vi "UHR-Fleezers Control (host) - 12.7c.vi"() -> ()   [LabVIEW 2012] (continued)
      }
      event "Abort AOD Scan": Value Change {
        n1196 = event-data() -> ()  [unwired: 7 out]
        n1197 = xnode "Read/Write Control"("FPGA VI Reference In"=w1678, "error in"=w1677, "Abort scan"="Abort AOD Scan") -> ("error out"=w1676:errorcluster)  [unwired: 1 out]
      }
      event "Continuous AOD Scanning": Value Change {
        n1198 = event-data() -> ()  [unwired: 7 out]
        n1199 = xnode "Read/Write Control"("FPGA VI Reference In"=w1682, "error in"=w1681, "Cont. Scan"="Continuous AOD Scanning") -> ("error out"=w1680:errorcluster)  [unwired: 1 out]
      }
      event "Index": Value Change {
        n1200 = event-data() -> ()  [unwired: 7 out]
        n1201 = call "Create new save file.vi"("Insert"="", "Ext"=".dat" ("string"), "Index In"="Index") -> ("Path Out"=→"Save file name":path, "Index Out"=w1683:dbl)
        "Save index" <- w1683
        n1202 = local write "Index"(w1683) -> ()
      }
      event "AO1", "AO2": Value Change {
        w1698 = 10.0 ("y")
        w1697 = 32767.0 ("y")
        n1203 = event-data() -> ()  [unwired: 7 out]
        n1204 = local read "AO2"() -> (w1696:dbl)
        n1205 = local read "AO1"() -> (w1693:dbl)
        n1206 = Multiply(x=w1693, y=w1697) -> (x*y=w1692:dbl)
        n1207 = Multiply(x=w1696, y=w1697) -> (x*y=w1695:dbl)
        n1208 = Divide(x=w1692, y=w1698) -> (x/y=w1691:dbl)
        n1209 = Divide(x=w1695, y=w1698) -> (x/y=w1694:dbl)
        n1210 = To Word Integer(number=w1691) -> (16bit integer=w1699:i16)
        n1211 = To Word Integer(number=w1694) -> (16bit integer=w1700:i16)
        n1212 = xnode "Read/Write Control"("FPGA VI Reference In"=w1690, "error in"=w1689, "AO1"=w1699, "AO2"=w1700) -> ("error out"=w1688:errorcluster)  [unwired: 1 out]
      }
      event "Inject Pump 1": Value Change {
        n1213 = event-data() -> ()  [unwired: 7 out]
        n1214 = local read "Use Harvard pumps\nfor beads (else Chemyx)"() -> (w1702:bool)
        n1215 = case shown="True" w1702 {
          tunnel: "Inject Pump 1" -> [w1706 w1744]
          tunnel: w1701 -> [_ w1745]
          frame False {
            n1216 = local read "Pump write delay (ms)"() -> (w1705:dbl)
            n1217 = local read "Chemyx Syringe Pump Serial Port"() -> (w1704:refnum<visa-resource-name>)
            n1218 = case shown="True" w1706 {
              tunnel: w1705 -> [w1712 w1726]
              tunnel: w1704 -> [w1709 w1725]
              frame False {
                n1219 = flat-sequence {
                  tunnel: w1709 -> [w1713]
                  tunnel: [w1713] -> w1710
                  tunnel: w1712 -> [_]
                  tunnel: [w1716] -> w1711
                  tunnel: w1710 -> [w1716]
                  tunnel: w1711 -> [w1717]
                  tunnel: [w1717] -> w1707
                  tunnel: [w1719] -> w1708
                  tunnel: w1707 -> [w1719]
                  tunnel: w1708 -> [w1721]
                  frame #0 {
                    n1220 = call "Write to pump.vi"("string"="enter pump1", "VISA resource name"=w1713) -> ()  [unwired: 1 out]
                  }
                  frame #1 {
                    n1221 = Wait (ms)(milliseconds to wait="Pump pause delay (ms)") -> ()  [unwired: 1 out]
                  }
                  frame #2 {
                    n1222 = call "Write to pump.vi"("string"="stop", "VISA resource name"=w1717) -> ()  [unwired: 1 out]
                  }
                  frame #3 {
                    n1223 = Wait (ms)(milliseconds to wait=u32 500) -> ()  [unwired: 1 out]
                  }
                  frame #4 {
                    n1224 = call "Write to pump.vi"("string"="stop", "VISA resource name"=w1721) -> ()  [unwired: 1 out]
                  }
                }
              }
              frame True {
                n1225 = flat-sequence {
                  tunnel: w1725 -> [w1735]
                  tunnel: w1726 -> [w1730]
                  tunnel: w1726 -> [w1737]
                  tunnel: w1725 -> [w1738]
                  tunnel: [w1738] -> w1723
                  tunnel: [w1740] -> w1724
                  tunnel: w1723 -> [w1740]
                  tunnel: w1724 -> [w1742]
                  frame #0 {
                    n1226 = local read "All Pump Parameters"() -> (w1729:T5)
                    n1227 = Unbundle By Name(w1729) -> ("Pump 1"=w1736:T30)
                    n1228 = call "Set pump parameters.vi"("Pump write delay (ms)"=w1730, "Volume (uL)"="Ch 1 Inject Volume (uL)", "Rate (uL/h)"="Ch 1 Inject Rate (ul/h)", "Units"=4.0, "Pump #"=1.0, "Pump Parameters In"=w1736, "VISA resource name"=w1735) -> ("Pump Parameters Out"=w1728:T30)  [unwired: 3 in]
                    n1229 = Bundle By Name(cluster=w1729, "Pump 1"=w1728) -> (w1727:T5)
                    n1230 = local write "All Pump Parameters"(w1727) -> ()
                  }
                  frame #1 {
                    n1231 = Wait (ms)(milliseconds to wait=w1737) -> ()  [unwired: 1 out]
                  }
                  frame #2 {
                    n1232 = call "Write to pump.vi"("string"="start", "VISA resource name"=w1738) -> ()  [unwired: 1 out]
                  }
                  frame #3 {
                    n1233 = Wait (ms)(milliseconds to wait=u32 500) -> ()  [unwired: 1 out]
                  }
                  frame #4 {
                    n1234 = call "Write to pump.vi"("string"="start", "VISA resource name"=w1742) -> ()  [unwired: 1 out]
                  }
                }
              }
            }
          }
          frame True {
            n1235 = case shown="False" w1744 {
              tunnel: w1745 -> [w1746 w1756]
              frame False {
                n1236 = flat-sequence {
                  tunnel: w1746 -> [w1748]
                  frame #0 {
                    n1237 = local write "Flushing P1"(FALSE ("Flushing P1")) -> ()
                    n1238 = Concatenate Strings("stop" ("string"), "\r") -> (w1750:string)
                    n1239 = VISA Write(VISA resource name=w1748, write buffer=w1750) -> ()  [unwired: 1 in, 3 out]
                  }
                  frame #1 {
                    n1240 = property on="Clear Volume P1" class="Bool (strict)"("Val(Sgnl)"=TRUE ("Value (Signaling)")) -> ()  [unwired: 2 in, 2 out]
                  }
                }
              }
              frame True {
                n1241 = local read "Normal Flow Rate (ul/h) P1"() -> (w1754:dbl)
                n1242 = Number To Decimal String(number=w1754) -> (decimal integer string=w1760:string)  [unwired: 1 in]
                n1243 = Concatenate Strings("irate  " ("string"), w1760, " u/h" ("string"), "\r") -> (w1758:string)
                n1244 = VISA Write(VISA resource name=w1756, write buffer=w1758) -> (VISA resource name out=w1755:refnum<visa-resource-name>)  [unwired: 1 in, 2 out]
                n1245 = Concatenate Strings("irun" ("string"), "\r") -> (w1762:string)
                n1246 = VISA Write(VISA resource name=w1755, write buffer=w1762) -> ()  [unwired: 1 in, 3 out]
              }
            }
          }
        }
      }
      event "Inject Pump 3": Value Change {
        n1247 = event-data() -> ()  [unwired: 7 out]
        n1248 = local read "Use Harvard pumps\nfor beads (else Chemyx)"() -> (w1765:bool)
        n1249 = case shown="True" w1765 {
          tunnel: "Inject Pump 3" -> [w1769 w1808]
          tunnel: w1764 -> [_ w1807]
          frame False {
            n1250 = local read "Pump write delay (ms)"() -> (w1768:dbl)
            n1251 = case shown="True" w1769 {
              tunnel: w1768 -> [w1775 w1789]
              tunnel: "Chemyx Syringe Pump Serial Port" -> [w1772 w1788]
              frame False {
                n1252 = flat-sequence {
                  tunnel: w1772 -> [w1776]
                  tunnel: [w1776] -> w1773
                  tunnel: w1775 -> [_]
                  tunnel: [w1779] -> w1774
                  tunnel: w1773 -> [w1779]
                  tunnel: w1774 -> [w1780]
                  tunnel: [w1780] -> w1770
                  tunnel: [w1782] -> w1771
                  tunnel: w1770 -> [w1782]
                  tunnel: w1771 -> [w1784]
                  frame #0 {
                    n1253 = call "Write to pump.vi"("string"="enter pump3", "VISA resource name"=w1776) -> ()  [unwired: 1 out]
                  }
                  frame #1 {
                    n1254 = local read "Pump pause delay (ms)"() -> (w1778:u32)
                    n1255 = Wait (ms)(milliseconds to wait=w1778) -> ()  [unwired: 1 out]
                  }
                  frame #2 {
                    n1256 = call "Write to pump.vi"("string"="stop", "VISA resource name"=w1780) -> ()  [unwired: 1 out]
                  }
                  frame #3 {
                    n1257 = Wait (ms)(milliseconds to wait=u32 0) -> ()  [unwired: 1 out]
                  }
                  frame #4 {
                    n1258 = call "Write to pump.vi"("string"="stop", "VISA resource name"=w1784) -> ()  [unwired: 1 out]
                  }
                }
              }
              frame True {
                n1259 = flat-sequence {
                  tunnel: w1788 -> [w1798]
                  tunnel: w1789 -> [w1793]
                  tunnel: w1789 -> [w1800]
                  tunnel: w1788 -> [w1801]
                  tunnel: [w1801] -> w1787
                  tunnel: [w1804] -> w1786
                  tunnel: w1787 -> [w1804]
                  tunnel: w1786 -> [w1805]
                  frame #0 {
                    n1260 = local read "All Pump Parameters"() -> (w1792:T5)
                    n1261 = Unbundle By Name(w1792) -> ("Pump 3"=w1799:T30)
                    n1262 = call "Set pump parameters.vi"("Pump write delay (ms)"=w1793, "Volume (uL)"="Ch 3 Inject Volume (uL)", "Rate (uL/h)"="Ch 3 Inject Rate (ul/h)", "Units"=4.0, "Pump #"=3.0, "Pump Parameters In"=w1799, "VISA resource name"=w1798) -> ("Pump Parameters Out"=w1791:T30)  [unwired: 3 in]
                    n1263 = Bundle By Name(cluster=w1792, "Pump 3"=w1791) -> (w1790:T5)
                    n1264 = local write "All Pump Parameters"(w1790) -> ()
                  }
                  frame #1 {
                    n1265 = Wait (ms)(milliseconds to wait=w1800) -> ()  [unwired: 1 out]
                  }
                  frame #2 {
                    n1266 = call "Write to pump.vi"("string"="start", "VISA resource name"=w1801) -> ()  [unwired: 1 out]
                  }
                  frame #3 {
                    n1267 = Wait (ms)(milliseconds to wait=u32 500) -> ()  [unwired: 1 out]
                  }
                  frame #4 {
                    n1268 = call "Write to pump.vi"("string"="start", "VISA resource name"=w1805) -> ()  [unwired: 1 out]
                  }
                }
              }
            }
          }
          frame True {
            n1269 = case shown="False" w1808 {
              tunnel: w1807 -> [w1809 w1816]
              frame False {
                n1270 = flat-sequence {
                  tunnel: w1809 -> [w1811]
                  frame #0 {
                    n1271 = local write "Flushing P3"(FALSE ("Flushing P3")) -> ()
                    n1272 = Concatenate Strings("stop" ("string"), "\r") -> (w1813:string)
                    n1273 = VISA Write(VISA resource name=w1811, write buffer=w1813) -> ()  [unwired: 1 in, 3 out]
                  }
                  frame #1 {
                    n1274 = property on="Clear Volume P3" class="Bool (strict)"("Val(Sgnl)"=TRUE ("Value (Signaling)")) -> ()  [unwired: 2 in, 2 out]
                  }
                }
              }
              frame True {
                n1275 = local read "Normal Flow Rate (ul/h) P3"() -> (w1817:dbl)
                n1276 = Number To Decimal String(number=w1817) -> (decimal integer string=w1823:string)  [unwired: 1 in]
                n1277 = Concatenate Strings("irate  " ("string"), w1823, " u/h" ("string"), "\r") -> (w1821:string)
                n1278 = VISA Write(VISA resource name=w1816, write buffer=w1821) -> (VISA resource name out=w1819:refnum<visa-resource-name>)  [unwired: 1 in, 2 out]
                n1279 = Concatenate Strings("irun" ("string"), "\r") -> (w1825:string)
                n1280 = VISA Write(VISA resource name=w1819, write buffer=w1825) -> ()  [unwired: 1 in, 3 out]
              }
            }
          }
        }
      }
      event "Inject Pump 2": Value Change {
        n1281 = event-data() -> ()  [unwired: 7 out]
        n1282 = local read "Pump write delay (ms)"() -> (w1829:dbl)
        n1283 = flat-sequence {
          tunnel: w1827 -> [w1842]
          tunnel: w1829 -> [w1838]
          tunnel: "Inject Pump 2" -> [_]
          tunnel: w1829 -> [w1844]
          tunnel: w1827 -> [w1845]
          frame #0 {
            n1284 = local read "All Pump Parameters"() -> (w1837:T5)
            n1285 = Multiply(x=60.0, y="Flush Center Ch Rate (ul/m)") -> (x*y=w1834:dbl)
            n1286 = Unbundle By Name(w1837) -> ("Pump 2"=w1843:T30)
            n1287 = call "Set pump parameters.vi"("Pump write delay (ms)"=w1838, "Volume (uL)"="Flush Center Ch Volume (uL)", "Rate (uL/h)"=w1834, "Units"=3.0, "Pump #"=2.0, "Pump Parameters In"=w1843, "VISA resource name"=w1842) -> ("Pump Parameters Out"=w1836:T30)  [unwired: 3 in]
            n1288 = Bundle By Name(cluster=w1837, "Pump 2"=w1836) -> (w1835:T5)
            n1289 = local write "All Pump Parameters"(w1835) -> ()
            n1290 = Add(x="Flush Center Ch Volume (uL)", y="Total Volume\nFlushed (uL)") -> (x+y=w1831:dbl)
            n1291 = local write "Total Volume\nFlushed (uL)"(w1831) -> ()
          }
          frame #1 {
            n1292 = Wait (ms)(milliseconds to wait=w1844) -> ()  [unwired: 1 out]
          }
          frame #2 {
            n1293 = call "Write to pump.vi"("string"="start", "VISA resource name"=w1845) -> ()  [unwired: 1 out]
          }
        }
        n1294 = local read "Chemyx Syringe Pump Serial Port"() -> (w1827:refnum<visa-resource-name>)
      }
      event "Sample Channel\nFlow": Value Change {
        n1295 = event-data() -> ()  [unwired: 7 out]
        n1296 = Select(t="irun" ("string"), s="Sample Channel\nFlow", f="stop" ("string")) -> (s? t:f=w1849:string)
        n1297 = Concatenate Strings(w1849, "\r") -> (w1852:string)
        n1298 = VISA Write(VISA resource name=w1847, write buffer=w1852) -> ()  [unwired: 1 in, 3 out]
      }
      event "Start Flow": Value Change {
        n1299 = event-data() -> ()  [unwired: 7 out]
        n1300 = local write "Sample Channel\nFlow"(TRUE ("Sample Channel\nFlow")) -> ()
        n1301 = local write "Start Flow"(FALSE ("Start Flow")) -> ()
        n1302 = Concatenate Strings("irun" ("string"), "\r") -> (w1858:string)
        n1303 = VISA Write(VISA resource name=w1854, write buffer=w1858) -> ()  [unwired: 1 in, 3 out]
      }
      event "Stop Flow": Value Change {
        w1860 = FALSE ("Stop Flow")
        n1304 = event-data() -> ()  [unwired: 7 out]
        n1305 = local write "Stop Flow"(w1860) -> ()
        n1306 = local write "Sample Channel\nFlow"(w1860) -> ()
        n1307 = Concatenate Strings("stop" ("string"), "\r") -> (w1863:string)
        n1308 = VISA Write(VISA resource name=w1861, write buffer=w1863) -> ()  [unwired: 1 in, 3 out]
      }
      event "Flow rate (uL/h)": Value Change {
        n1309 = event-data() -> ()  [unwired: 7 out]
        n1310 = Number To Decimal String(number="Flow rate (uL/h)") -> (decimal integer string=w1870:string)  [unwired: 1 in]
        n1311 = Concatenate Strings("irate  " ("string"), w1870, " u/h" ("string"), "\r") -> (w1869:string)
        n1312 = VISA Write(VISA resource name=w1866, write buffer=w1869) -> ()  [unwired: 1 in, 3 out]
      }
      event "Flush Sample": Value Change {
        n1313 = event-data() -> ()  [unwired: 7 out]
        n1314 = flat-sequence {
          tunnel: w1875 -> [w1903]
          tunnel: [w1883] -> w1874
          tunnel: [w1877] -> w1872
          tunnel: w1874 -> [w1907]
          tunnel: [w1907] -> w1873
          tunnel: w1872 -> [w1906]
          tunnel: w1873 -> [w1912]
          frame #0 {
            # "set paramaters (rate, volume) for flush, clear volume"
            n1315 = Number To Decimal String(number="Flush rate (uL/m)") -> (decimal integer string=w1899:string)  [unwired: 1 in]
            n1316 = Concatenate Strings("irate  " ("string"), w1899, " u/m" ("string"), "\r") -> (w1901:string)
            n1317 = VISA Write(VISA resource name=w1903, write buffer=w1901) -> (VISA resource name out=w1897:refnum<visa-resource-name>)  [unwired: 1 in, 2 out]
            n1318 = Reciprocal(x="Flush rate (uL/m)") -> (1/x=w1880:dbl)
            n1319 = Number To Decimal String(number="Volume (uL)") -> (decimal integer string=w1888:string)  [unwired: 1 in]
            n1320 = Multiply(x="Volume (uL)", y=w1880) -> (x*y=w1879:dbl)
            n1321 = Concatenate Strings("tvolume  " ("string"), w1888, " u" ("string"), "\r") -> (w1886:string)
            n1322 = Multiply(x=w1879, y=60000.0) -> (x*y=w1877:dbl)
            n1323 = VISA Write(VISA resource name=w1897, write buffer=w1886) -> (VISA resource name out=w1885:refnum<visa-resource-name>)  [unwired: 1 in, 2 out]
            n1324 = Concatenate Strings("cvolume" ("string"), "\r") -> (w1884:string)
            n1325 = VISA Write(VISA resource name=w1885, write buffer=w1884) -> (VISA resource name out=w1895:refnum<visa-resource-name>)  [unwired: 1 in, 2 out]
            n1326 = Concatenate Strings("irun" ("string"), "\r") -> (w1893:string)
            n1327 = VISA Write(VISA resource name=w1895, write buffer=w1893) -> (VISA resource name out=w1883:refnum<visa-resource-name>)  [unwired: 1 in, 2 out]
          }
          frame #1 {
            # "Have to wait until\nflow is done to reset\nrate"
            n1328 = Add(x=w1906, y=100.0) -> (x+y=w1905:dbl)
            n1329 = Wait (ms)(milliseconds to wait=w1905) -> ()  [unwired: 1 out]
          }
          frame #2 {
            # "reset flow rate to usual flow rate"
            n1330 = local read "Flow rate (uL/h)"() -> (w1918:dbl)
            n1331 = Number To Decimal String(number=w1918) -> (decimal integer string=w1916:string)  [unwired: 1 in]
            n1332 = Concatenate Strings("irate  " ("string"), w1916, " u/h" ("string"), "\r") -> (w1914:string)
            n1333 = VISA Write(VISA resource name=w1912, write buffer=w1914) -> (VISA resource name out=w1908:refnum<visa-resource-name>)  [unwired: 1 in, 2 out]
            n1334 = Concatenate Strings("cvolume" ("string"), "\r") -> (w1909:string)
            n1335 = VISA Write(VISA resource name=w1908, write buffer=w1909) -> ()  [unwired: 1 in, 3 out]
          }
        }
      }
      event "Flush Pump 3": Value Change {
        n1336 = event-data() -> ()  [unwired: 7 out]
        n1337 = flat-sequence {
          tunnel: w1919 -> [w1922]
          frame #0 {
            # "set paramaters (rate, volume) for flush, clear volume"
            n1338 = Number To Decimal String(number="Flush rate (uL/m) P3") -> (decimal integer string=w1944:string)  [unwired: 1 in]
            n1339 = local write "Inject Pump 3"(TRUE ("Inject Pump 3")) -> ()
            n1340 = Concatenate Strings("irate  " ("string"), w1944, " u/m" ("string"), "\r") -> (w1946:string)
            n1341 = VISA Write(VISA resource name=w1922, write buffer=w1946) -> (VISA resource name out=w1942:refnum<visa-resource-name>)  [unwired: 1 in, 2 out]
            n1342 = Reciprocal(x="Flush rate (uL/m) P3") -> (1/x=w1926:dbl)
            n1343 = Number To Decimal String(number="Volume (uL) P3") -> (decimal integer string=w1933:string)  [unwired: 1 in]
            n1344 = Multiply(x="Volume (uL) P3", y=w1926) -> (x*y=w1925:dbl)
            n1345 = Concatenate Strings("tvolume  " ("string"), w1933, " u" ("string"), "\r") -> (w1931:string)
            n1346 = Multiply(x=w1925, y=60.0) -> (x*y=→"HP3 Flush Time (s)":dbl)
            n1347 = VISA Write(VISA resource name=w1942, write buffer=w1931) -> (VISA resource name out=w1930:refnum<visa-resource-name>)  [unwired: 1 in, 2 out]
            n1348 = Concatenate Strings("cvolume" ("string"), "\r") -> (w1929:string)
            n1349 = VISA Write(VISA resource name=w1930, write buffer=w1929) -> (VISA resource name out=w1940:refnum<visa-resource-name>)  [unwired: 1 in, 2 out]
            n1350 = Concatenate Strings("irun" ("string"), "\r") -> (w1938:string)
            n1351 = VISA Write(VISA resource name=w1940, write buffer=w1938) -> ()  [unwired: 1 in, 3 out]
          }
          frame #1 {
            "Flushing P3" <- TRUE ("Flushing P3")
          }
        }
      }
      event "Flush Pump 1": Value Change {
        n1352 = event-data() -> ()  [unwired: 7 out]
        n1353 = flat-sequence {
          tunnel: [w1960] -> w1950
          tunnel: w1949 -> [w1953]
          tunnel: w1950 -> [_]
          frame #0 {
            # "set paramaters (rate, volume) for flush, clear volume"
            n1354 = local write "Inject Pump 1"(TRUE ("Inject Pump 1")) -> ()
            n1355 = Number To Decimal String(number="Flush rate (uL/m) P1") -> (decimal integer string=w1976:string)  [unwired: 1 in]
            n1356 = Concatenate Strings("irate  " ("string"), w1976, " u/m" ("string"), "\r") -> (w1978:string)
            n1357 = VISA Write(VISA resource name=w1953, write buffer=w1978) -> (VISA resource name out=w1974:refnum<visa-resource-name>)  [unwired: 1 in, 2 out]
            n1358 = Reciprocal(x="Flush rate (uL/m) P1") -> (1/x=w1957:dbl)
            n1359 = Number To Decimal String(number="Volume (uL) P1") -> (decimal integer string=w1965:string)  [unwired: 1 in]
            n1360 = Multiply(x="Volume (uL) P1", y=w1957) -> (x*y=w1956:dbl)
            n1361 = Concatenate Strings("tvolume  " ("string"), w1965, " u" ("string"), "\r") -> (w1963:string)
            n1362 = Multiply(x=w1956, y=60.0) -> (x*y=→"HP1 Flush Time (s)":dbl)
            n1363 = VISA Write(VISA resource name=w1974, write buffer=w1963) -> (VISA resource name out=w1962:refnum<visa-resource-name>)  [unwired: 1 in, 2 out]
            n1364 = Concatenate Strings("cvolume" ("string"), "\r") -> (w1961:string)
            n1365 = VISA Write(VISA resource name=w1962, write buffer=w1961) -> (VISA resource name out=w1972:refnum<visa-resource-name>)  [unwired: 1 in, 2 out]
            n1366 = Concatenate Strings("irun" ("string"), "\r") -> (w1970:string)
            n1367 = VISA Write(VISA resource name=w1972, write buffer=w1970) -> (VISA resource name out=w1960:refnum<visa-resource-name>)  [unwired: 1 in, 2 out]
          }
          frame #1 {
            "Flushing P1" <- TRUE ("Flushing P3")
          }
        }
      }
      event "Clear Volume": Value Change {
        n1368 = event-data() -> ()  [unwired: 7 out]
        n1369 = Concatenate Strings("cvolume" ("string"), "\r") -> (w1982:string)
        n1370 = VISA Write(VISA resource name=w1981, write buffer=w1982) -> ()  [unwired: 1 in, 3 out]
      }
      event "Clear Volume P3": Value Change {
        n1371 = event-data() -> ()  [unwired: 7 out]
        n1372 = Concatenate Strings("cvolume" ("string"), "\r") -> (w1988:string)
        n1373 = VISA Write(VISA resource name=w1987, write buffer=w1988) -> ()  [unwired: 1 in, 3 out]
        n1374 = local write "Clear Volume P3"(FALSE ("Clear Volume P3")) -> ()
      }
      event "Clear Volume P1": Value Change {
        n1375 = event-data() -> ()  [unwired: 7 out]
        n1376 = Concatenate Strings("cvolume" ("string"), "\r") -> (w1993:string)
        n1377 = local write "Clear Volume P1"(FALSE ("Clear Volume P1")) -> ()
        n1378 = VISA Write(VISA resource name=w1992, write buffer=w1993) -> ()  [unwired: 1 in, 3 out]
      }
      event "Display On P3": Value Change {
        n1379 = event-data() -> ()  [unwired: 7 out]
        n1380 = Select(t="dim 100", s="Display On P3", f="dim 0") -> (s? t:f=w1999:string)
        n1381 = Concatenate Strings(w1999, "\r") -> (w2001:string)
        n1382 = VISA Write(VISA resource name=w1996, write buffer=w2001) -> ()  [unwired: 1 in, 3 out]
      }
      event "Display On P1": Value Change {
        n1383 = event-data() -> ()  [unwired: 7 out]
        n1384 = Select(t="dim 100", s="Display On P1", f="dim 0") -> (s? t:f=w2006:string)
        n1385 = Concatenate Strings(w2006, "\r") -> (w2008:string)
        n1386 = VISA Write(VISA resource name=w2003, write buffer=w2008) -> ()  [unwired: 1 in, 3 out]
      }
      event "Retract Pump 3": Value Change {
        n1387 = event-data() -> ()  [unwired: 7 out]
        n1388 = local write "Retract Pump 3"(FALSE ("Retract Pump 3")) -> ()
        n1389 = case shown="True" "Retract Pump 3" {
          tunnel: w2010 -> [_ w2013]
          frame False {
          }
          frame True {
            n1390 = Number To Decimal String(number="Retract Rate (uL/m)") -> (decimal integer string=w2031:string)  [unwired: 1 in]
            n1391 = Concatenate Strings("wrate  " ("string"), w2031, " u/m" ("string"), "\r") -> (w2033:string)
            n1392 = VISA Write(VISA resource name=w2013, write buffer=w2033) -> (VISA resource name out=w2024:refnum<visa-resource-name>)  [unwired: 1 in, 2 out]
            n1393 = Number To Decimal String(number="Retract Vol 3 (uL)") -> (decimal integer string=w2026:string)  [unwired: 1 in]
            n1394 = Concatenate Strings("tvolume  " ("string"), w2026, " u" ("string"), "\r") -> (w2023:string)
            n1395 = VISA Write(VISA resource name=w2024, write buffer=w2023) -> (VISA resource name out=w2019:refnum<visa-resource-name>)  [unwired: 1 in, 2 out]
            n1396 = Concatenate Strings("cvolume" ("string"), "\r") -> (w2020:string)
            n1397 = VISA Write(VISA resource name=w2019, write buffer=w2020) -> (VISA resource name out=w2014:refnum<visa-resource-name>)  [unwired: 1 in, 2 out]
            n1398 = Concatenate Strings("wrun" ("string"), "\r") -> (w2015:string)
            n1399 = VISA Write(VISA resource name=w2014, write buffer=w2015) -> ()  [unwired: 1 in, 3 out]
          }
        }
      }
      event "Retract Pump 1": Value Change {
        n1400 = event-data() -> ()  [unwired: 7 out]
        n1401 = local write "Retract Pump 1"(FALSE ("Retract Pump 1")) -> ()
        n1402 = case shown="True" "Retract Pump 1" {
          tunnel: w2035 -> [_ w2040]
          frame False {
          }
          frame True {
            n1403 = local read "Retract Rate (uL/m)"() -> (w2038:dbl)
            n1404 = Number To Decimal String(number=w2038) -> (decimal integer string=w2056:string)  [unwired: 1 in]
            n1405 = Concatenate Strings("wrate  " ("string"), w2056, " u/m" ("string"), "\r") -> (w2058:string)
            n1406 = VISA Write(VISA resource name=w2040, write buffer=w2058) -> (VISA resource name out=w2050:refnum<visa-resource-name>)  [unwired: 1 in, 2 out]
            n1407 = Number To Decimal String(number="Retract Vol 1 (uL)") -> (decimal integer string=w2052:string)  [unwired: 1 in]
            n1408 = Concatenate Strings("tvolume  " ("string"), w2052, " u" ("string"), "\r") -> (w2049:string)
            n1409 = VISA Write(VISA resource name=w2050, write buffer=w2049) -> (VISA resource name out=w2046:refnum<visa-resource-name>)  [unwired: 1 in, 2 out]
            n1410 = Concatenate Strings("cvolume" ("string"), "\r") -> (w2047:string)
            n1411 = VISA Write(VISA resource name=w2046, write buffer=w2047) -> (VISA resource name out=w2041:refnum<visa-resource-name>)  [unwired: 1 in, 2 out]
            n1412 = Concatenate Strings("wrun" ("string"), "\r") -> (w2042:string)
            n1413 = VISA Write(VISA resource name=w2041, write buffer=w2042) -> ()  [unwired: 1 in, 3 out]
          }
        }
      }
      event "Flip Green Filter": Value Change {
        n1414 = event-data() -> ()  [unwired: 7 out]
        n1415 = Not(x="Flip Green Filter") -> (.not. x?=w2060:bool)
        n1416 = local write "Flip Green Filter"(w2060) -> ()
        n1417 = flat-sequence {
          tunnel: w2068 -> [w2073]
          tunnel: w2067 -> [w2072]
          tunnel: [w2070] -> w2065
          tunnel: [w2069] -> w2064
          tunnel: [w2075] -> w2063
          tunnel: w2065 -> [w2075]
          tunnel: [w2074] -> w2062
          tunnel: w2064 -> [w2074]
          tunnel: w2063 -> [w2079]
          tunnel: w2062 -> [w2078]
          tunnel: [w2077] -> w2066
          frame #0 {
            n1418 = xnode "Read/Write Control"("FPGA VI Reference In"=w2073, "error in"=w2072, "Green Filter Flipper"=TRUE) -> ("FPGA VI Reference Out"=w2070:T20, "error out"=w2069:errorcluster)
          }
          frame #1 {
            n1419 = Wait (ms)(milliseconds to wait=u32 100) -> ()  [unwired: 1 out]
          }
          frame #2 {
            n1420 = xnode "Read/Write Control"("FPGA VI Reference In"=w2079, "error in"=w2078, "Green Filter Flipper"=FALSE) -> ("error out"=w2077:errorcluster)  [unwired: 1 out]
          }
        }
      }
      event "Pump 1 contents", "Pump 3 contents": Value Change {
        n1421 = event-data() -> ()  [unwired: 7 out]
        n1422 = local read "Pump 1 contents"() -> (→"Pump 1 cont disp":string)
        n1423 = local read "Pump 3 contents"() -> (→"Pump 3 cont disp":string)
      }
      event "Reset Trap Pos. FB": Value Change {
        n1424 = event-data() -> ()  [unwired: 7 out]
        n1425 = xnode "Read/Write Control"("FPGA VI Reference In"=w2085, "error in"=w2084, "Trap Pos. FB Reset"="Reset Trap Pos. FB") -> ()  [unwired: 2 out]
      }
      event "Rem fb disp offset": Value Change {
        n1426 = event-data() -> ()  [unwired: 7 out]
        n1427 = local write "Rem fb disp offset"(FALSE ("Rem fb disp offset")) -> ()
        n1428 = local read "Mean T1 Position (nm)"() -> (w2087:dbl)
        n1429 = local read "FB Trap Pos Offset"() -> (w2088:dbl)
        n1430 = Subtract(x=w2088, y=w2087) -> (x-y=w2086:dbl)
        n1431 = local write "FB Trap Pos Offset"(w2086) -> ()
      }
      event "Threshold (nm)": Value Change {
        n1432 = event-data() -> ()  [unwired: 7 out]
        n1433 = flat-sequence {
          tunnel: w2092 -> [w2100]
          tunnel: w2091 -> [w2099]
          tunnel: [w2093] -> w2090
          tunnel: w2090 -> [w2106]
          frame #0 {
            n1434 = xnode "Read/Write Control"("FPGA VI Reference In"=w2100, "error in"=w2099) -> ("FPGA VI Reference Out"=w2096:T20, "error out"=w2095:errorcluster, "FPGA TTrig Thresh"=w2097:i64)
            n1435 = local read "Threshold stored (nm)"() -> (w2105:dbl)
            n1436 = local read "Threshold (nm)"() -> (w2093:dbl)
            n1437 = local read "AOM X Cal (nm/MHz)"() -> (w2103:dbl)
            n1438 = Subtract(x=w2093, y=w2105) -> (x-y=w2104:dbl)
            n1439 = Divide(x=w2104, y=w2103) -> (x/y=w2101:dbl)
            n1440 = call "IR AOM freq to word.vi"("Frequency In (MHz)"=w2101) -> ("Frequency Word Out (double)"=w2102:dbl)
            n1441 = To Quad Integer(1:w2102) -> (0:w2098:i64)
            n1442 = Add(x=w2097, y=w2098) -> (x+y=w2094:i64)
            n1443 = xnode "Read/Write Control"("FPGA VI Reference In"=w2096, "error in"=w2095, "FPGA TTrig Thresh"=w2094) -> ()  [unwired: 2 out]
          }
          frame #1 {
            "Threshold stored (nm)" <- w2106
          }
        }
      }
      event "FB Trig Integrate": Value Change {
        n1444 = event-data() -> ()  [unwired: 7 out]
        n1445 = local read "FB Trig Integrate"() -> (w2108:u32)
        n1446 = xnode "Read/Write Control"("FPGA VI Reference In"=w2110, "error in"=w2109, "FB Trig Integrate"=w2108) -> ("error out"=w2107:errorcluster)  [unwired: 1 out]
      }
      event "11": Value Change {
        n1447 = event-data() -> ()  [unwired: 7 out]
        n1448 = local read "11"() -> (w2111:bool)
        n1449 = case shown="True" w2111 {
          frame False {
          }
          frame True {
            n1450 = local read "Messages"() -> (w2113:string)
            n1451 = call "Update messages.vi"("Message to add"="You kicked it up to 11!", "Old message string"=w2113) -> ("New message string"=w2114:string)
            n1452 = call <vilib>:"Beep.vi"() -> ()  [unwired: 12 in]
            n1453 = local write "Messages"(w2114) -> ()
          }
        }
      }
      event "Trap Pos. FB ON": Value Change {
        n1454 = event-data() -> ()  [unwired: 7 out]
        n1455 = xnode "Read/Write Control"("FPGA VI Reference In"=w2117, "error in"=w2116, "Force feedback"="Trap Pos. FB ON") -> ()  [unwired: 2 out]
      }
      event "Remove Action Offset": Value Change {
        n1456 = event-data() -> ()  [unwired: 7 out]
        n1457 = local write "Remove Action Offset"(FALSE ("Remove Action Offset")) -> ()
        n1458 = local read "Trap Pos. FB Mult Factor"() -> (w2122:i64)
        n1459 = local read "Trap Pos FB Action"() -> (w2120:i64)
        n1460 = local read "Trap Pos. FB Offset Factor"() -> (w2118:i64)
        n1461 = Multiply(x=w2122, y=w2120) -> (x*y=w2121:i64)
        n1462 = Add(x=w2121, y=w2118) -> (x+y=w2119:i64)
        n1463 = local write "Trap Pos. FB Offset Factor"(w2119) -> ()
        n1464 = xnode "Read/Write Control"("FPGA VI Reference In"=w2125, "error in"=w2124, "Trap Pos. FB Offset Factor"=w2119) -> ()  [unwired: 2 out]
      }
      event "Remove Unwinding Offset": Value Change {
        n1465 = event-data() -> ()  [unwired: 7 out]
        n1466 = local write "Remove Unwinding Offset"(FALSE ("Remove Action Offset")) -> ()
        n1467 = local read "Trap Pos. FB Mult Factor"() -> (w2137:i64)
        n1468 = local read "Trap Pos FB Action"() -> (w2135:i64)
        n1469 = local read "Trap Pos. FB Offset Factor"() -> (w2134:i64)
        n1470 = Multiply(x=w2137, y=w2135) -> (x*y=w2136:i64)
        n1471 = local read "Trap Pos. FB Mult Factor"() -> (w2133:i64)
        n1472 = Add(x=w2136, y=w2134) -> (x+y=w2127:i64)
        n1473 = Multiply(x=32768, y="factor") -> (x*y=w2130:dbl)
        n1474 = Multiply(x=w2130, y=w2133) -> (x*y=w2132:dbl)
        n1475 = Subtract(x=w2127, y=w2132) -> (x-y=w2131:dbl)
        n1476 = To Quad Integer(1:w2131) -> (0:w2126:i64)
        n1477 = xnode "Read/Write Control"("FPGA VI Reference In"=w2140, "error in"=w2139, "Trap Pos. FB Offset Factor"=w2126) -> ()  [unwired: 2 out]
        n1478 = local write "Trap Pos. FB Offset Factor"(w2126) -> ()
      }
      event "Trap Pos. FB Range", "Trap Pos. FB Gains", "Trap Pos. FB Mult Factor", "Trap Pos. FB Offset Factor", "Trap Pos FB Negate Action", "Trap Pos FB Monitor\nT1 or T2", "Differential FB?", "Negate Diff?": Value Change {
        n1479 = event-data() -> ()  [unwired: 7 out]
        n1480 = Unbundle By Name("Trap Pos. FB Gains") -> ("proportional gain (Kc)"=w2143:fxp<+/-,16,8>, "integral gain (Kc*Ts/Ti)"=w2142:fxp<+/-,16,8>, "derivative gain (Kc*Td/Ts)"=w2141:fxp<+/-,16,8>)
        n1481 = local read "Negate Diff?"() -> (w2148:bool)
        n1482 = Unbundle By Name("Trap Pos. FB Range") -> ("output high"=w2146:fxp<+/-,16,1>, "output low"=w2145:fxp<+/-,16,1>)
        n1483 = xnode "Read/Write Control"("FPGA VI Reference In"=w2156, "error in"=w2155, "FB2 output high"=w2146, "FB2 output low"=w2145, "P2"=w2143, "I2"=w2142, "D2"=w2141, "Trap Pos. FB Mult Factor"="Trap Pos. FB Mult Factor", "Trap Pos. FB Offset Factor"="Trap Pos. FB Offset Factor", "Trap Pos FB Negate Action"="Trap Pos FB Negate Action", "Trap Pos FB Monitor T1 or T2"="Trap Pos FB Monitor\nT1 or T2", "AI1 X Scale"="Trap Pos. AI1 X Pre-scale", "Negate Diff?"=w2148, "Diff FB Measurement?"="Differential FB?") -> ()  [unwired: 2 out]
      }
      event "Trap Pos FB SP", "Trap Pos FB SP 2", "Use SP 2": Value Change {
        n1484 = event-data() -> ()  [unwired: 7 out]
        n1485 = Select(t="Trap Pos FB SP 2", s="Use SP 2", f="Trap Pos FB SP") -> (s? t:f=w2157:fxp<+/-,16,1>)
        n1486 = xnode "Read/Write Control"("FPGA VI Reference In"=w2162, "error in"=w2161, "Trap Pos. FB SP"=w2157) -> ()  [unwired: 2 out]
      }
      event "Offset SP2 from SP1": Value Change {
        n1487 = event-data() -> ()  [unwired: 7 out]
        n1488 = local read "Trap Pos FB SP"() -> (w2165:fxp<+/-,16,1>)
        n1489 = Add(x=w2165, y="SP2 Offset") -> (x+y=w2163:fxp<+/-,16,1>)
        n1490 = property on="Trap Pos FB SP 2" class="DigNum (strict)"("Val(Sgnl)"=w2163) -> ()  [unwired: 2 in, 2 out]
        n1491 = local write "Offset SP2 from SP1"(FALSE ("Offset SP2 from SP1")) -> ()
      }
      event "Set Reading to\nSetpoint": Value Change {
        # "This is the actual PID input signal"
        n1492 = event-data() -> ()  [unwired: 7 out]
        n1493 = local write "Set Reading to\nSetpoint"(FALSE ("Set SP to Reading")) -> ()
        n1494 = xnode "Read/Write Control"("FPGA VI Reference In"=w2171, "error in"=w2170) -> ("FPGA VI Reference Out"=w2169:T20, "error out"=w2168:errorcluster, "Trap Pos FB Int-Norm Signal"=w2167:fxp<+/-,16,1>)
        n1495 = local read "Differential FB?"() -> (w2172:bool)
        n1496 = case shown="False" w2172 {
          tunnel: [w2177 w2184] -> w2174
          tunnel: w2167 -> [w2175 w2184]
          frame False {
            n1497 = local read "Trap Pos FB Monitor\nT1 or T2"() -> (w2180:bool)
            n1498 = local read "Trap X AI1 (DMA)"() -> (w2183:T13)
            n1499 = Unbundle By Name(w2183) -> ("Set 1"=w2182:fxp<+/-,16,1>, "Set 2"=w2181:fxp<+/-,16,1>)
            n1500 = Select(t=w2182, s=w2180, f=w2181) -> (s? t:f=w2179:fxp<+/-,16,1>)
            n1501 = Not(x="Set SP Using...") -> (.not. x?=w2176:bool)
            n1502 = Select(t=w2175, s=w2176, f=w2179) -> (s? t:f=w2177:fxp<+/-,16,1>)
          }
          frame True {
          }
        }
        n1503 = xnode "Read/Write Control"("FPGA VI Reference In"=w2169, "error in"=w2168, "Trap Pos. FB SP"=w2174) -> ()  [unwired: 2 out]
        n1504 = local write "Trap Pos FB SP"(w2174) -> ()
      }
      event "Trap Pos. FB Out Scale 2^n": Value Change {
        n1505 = event-data() -> ()  [unwired: 7 out]
        n1506 = Scale By Power Of 2(n="Trap Pos. FB Out Scale 2^n", x=ext 1.0) -> (x*2^n=w2185:ext)
        n1507 = property on="Trap Pos. FB Mult Factor" class="DigNum (strict)"("Val(Sgnl)"=w2185) -> ()  [unwired: 2 in, 2 out]
      }
      event "Trap Pos FB Int Count": Value Change {
        n1508 = event-data() -> ()  [unwired: 7 out]
        n1509 = xnode "Read/Write Control"("FPGA VI Reference In"=w2190, "error in"=w2189, "Trap Pos FB Int Count"="Trap Pos FB Int Count") -> ()  [unwired: 2 out]
      }
      event "Trap pos": Value Change {
        n1510 = event-data() -> ()  [unwired: 7 out]
        n1511 = case shown="True" "Trap pos" {
          frame False {
            n1512 = property on="Trap Delta Graph" class="WFGraph (strict)"("Visible"=TRUE) -> ()  [unwired: 2 in, 2 out]
            n1513 = property on="Saved trap pos" class="WFGraph (strict)"("Visible"=FALSE) -> ()  [unwired: 2 in, 2 out]
          }
          frame True {
            n1514 = property on="Saved trap pos" class="WFGraph (strict)"("Visible"=TRUE) -> ()  [unwired: 2 in, 2 out]
            n1515 = property on="Trap Delta Graph" class="WFGraph (strict)"("Visible"=FALSE) -> ()  [unwired: 2 in, 2 out]
          }
        }
      }
    }
    "error out 2" <- w1011
    n1516 = node-c288() -> ()  [unwired: 2 out]
  }
  n1517 = timed-loop "Rough control of MCL mirror stage (debugging)" {
    tunnel: w1 -> [w2198]
    tunnel: [w2197] -> w261
    timing: w18 -> [_]
    timing-out: [_] -> w17
    stop <- w2197 stop-if-true
    n1518 = node-c288() -> ()  [unwired: 2 out]
    n1519 = case shown="1" "MCL Mode" {
      tunnel: w2198 -> [_ w2201 w2248]
      frame 0, Default {
      }
      frame 1 {
        n1520 = node-c288() -> (w2203:T23)  [unwired: 4 out]
        n1521 = timed-loop "Oscillate MCL mirror" {
          timing: w2203 -> [_]
          timing-out: [_] -> w2202
          tunnel: w2201 -> [w2242]
          i -> [w2241]
          stop <- w2204 stop-if-true
          n1522 = node-c288() -> (w2240:i64)  [unwired: 1 out]
          n1523 = Multiply(x="AO1", y=32767.0) -> (x*y=w2236:dbl)
          n1524 = Multiply(x="AO2", y=32767.0) -> (x*y=w2231:dbl)
          n1525 = Divide(x=w2236, y=10.0) -> (x/y=w2237:dbl)
          n1526 = Divide(x=w2231, y=10.0) -> (x/y=w2232:dbl)
          n1527 = To Word Integer(number=w2237) -> (16bit integer=w2229:i16)
          n1528 = To Word Integer(number=w2232) -> (16bit integer=w2228:i16)
          n1529 = Divide(x=w2240, y=i64 1000) -> (x/y=w2211:dbl)
          n1530 = Multiply(x=w2211, y=w2241) -> (x*y=w2222:dbl)
          n1531 = Multiply(x="Osc. freq. (Hz) 2", y=6.283185307179586) -> (x*y=w2223:dbl)
          n1532 = Multiply(x=w2223, y=w2222) -> (x*y=w2221:dbl)
          n1533 = Sine(x=w2221) -> (sin(x)=w2220:dbl)
          n1534 = Multiply(x=w2220, y="Osc. amp. (V)") -> (x*y=w2218:dbl)
          n1535 = Add(x=w2218, y="Osc. center (V)") -> (x+y=w2216:dbl)
          n1536 = Divide(x=w2216, y=10.0) -> (x/y=w2214:dbl)
          n1537 = Multiply(x=w2214, y=32767.0) -> (x*y=w2209:dbl)
          n1538 = Select(t=w2209, s="Scan axis", f=w2229) -> (s? t:f=w2227:dbl)
          n1539 = Select(t=w2228, s="Scan axis", f=w2209) -> (s? t:f=w2226:dbl)
          n1540 = local read "MCL Mode"() -> (w2208:u16)
          n1541 = Not Equal?(x=w2208, y=u16 1) -> (x != y?=w2205:bool)
          n1542 = local read "Stop All"() -> (w2206:bool)
          n1543 = xnode "Read/Write Control"("FPGA VI Reference In"=w2242, "AO1"=w2227, "AO2"=w2226) -> ()  [unwired: 1 in, 2 out]
          n1544 = Compound Arithmetic op=OR(w2206, w2205) -> (w2204:bool)
          n1545 = node-c288() -> ()  [unwired: 2 out]
        }
        n1546 = node-c288(w2202) -> ()  [unwired: 1 out]
      }
      frame 2 {
        n1547 = case shown="True" "Start Scan" {
          tunnel: w2248 -> [_ w2260]
          frame False {
          }
          frame True {
            n1548 = Subtract(x="End (V)", y="Begin (V)") -> (x-y=w2256:dbl)
            n1549 = Decrement(x="N Points") -> (x-1=w2255:dbl)
            n1550 = Divide(x=w2256, y=w2255) -> (x/y=w2253:dbl)
            n1551 = for {
              N: "N Points" -> [_]
              tunnel: "Begin (V)" -> [w2273]
              tunnel: w2260 -> [w2265]
              tunnel: [w2264] -> w2259 mode=indexing
              tunnel: w2253 -> [w2263]
              tunnel: [w2261] -> w2252 mode=indexing
              i -> [w2272]
              n1552 = Multiply(x=w2263, y=w2272) -> (x*y=w2271:dbl)
              n1553 = Add(x=w2273, y=w2271) -> (x+y=w2268:dbl)
              n1554 = local read "Scan axis"() -> (w2262:bool)
              n1555 = local read "AO1"() -> (w2270:dbl)
              n1556 = local read "AO2"() -> (w2269:dbl)
              n1557 = Select(t=w2268, s=w2262, f=w2270) -> (s? t:f=w2267:dbl)
              n1558 = Select(t=w2269, s=w2262, f=w2268) -> (s? t:f=w2266:dbl)
              n1559 = flat-sequence {
                tunnel: w2267 -> [w2277]
                tunnel: w2266 -> [w2276]
                tunnel: w2265 -> [w2274]
                tunnel: [w2287] -> w2264
                tunnel: [w2286] -> w2261
                frame #0 {
                  w2280 = 10.0 ("y")
                  w2275 = 32767.0 ("y")
                  n1560 = Multiply(x=w2277, y=w2275) -> (x*y=w2283:dbl)
                  n1561 = Multiply(x=w2276, y=w2275) -> (x*y=w2281:dbl)
                  n1562 = Divide(x=w2283, y=w2280) -> (x/y=w2284:dbl)
                  n1563 = Divide(x=w2281, y=w2280) -> (x/y=w2282:dbl)
                  n1564 = To Word Integer(number=w2284) -> (16bit integer=w2278:i16)
                  n1565 = To Word Integer(number=w2282) -> (16bit integer=w2279:i16)
                  n1566 = xnode "Read/Write Control"("FPGA VI Reference In"=w2274, "AO1"=w2278, "AO2"=w2279) -> ()  [unwired: 1 in, 2 out]
                }
                frame #1 {
                  n1567 = Wait (ms)(milliseconds to wait="DAQ Delay (ms)") -> ()  [unwired: 1 out]
                }
                frame #2 {
                  n1568 = local read "Slow mean"() -> (w2287:dbl)
                  n1569 = local read "Sigma"() -> (w2286:dbl)
                }
              }
            }
            n1570 = Bundle("Begin (V)"="Begin (V)", w2253, w2259) -> (→"MCL Scan":cluster{"Begin (V)":dbl, dbl, dbl[]})  [unwired: 1 out]
            n1571 = Bundle("Begin (V)"="Begin (V)", w2253, w2252) -> (→"MCL Scan 2":cluster{"Begin (V)":dbl, dbl, dbl[]})  [unwired: 1 out]
          }
        }
      }
    }
    n1572 = local read "Stop All"() -> (w2197:bool)
    n1573 = node-c288() -> ()  [unwired: 2 out]
  }
  n1574 = timed-loop "Mouse control: trap position (AOM deflection), set confocal spot from image" {
    tunnel: [w2289] -> w213
    tunnel: w1 -> [w2288]
    timing: w135 -> [_]
    timing-out: [_] -> w134
    stop <- w2289 stop-if-true
    n1575 = node-c288() -> ()  [unwired: 2 out]
    n1576 = event shown="[0] \"Pane\": Mouse Down" {
      selector: _ -> [_ _]
      dyn-events: _ -> [_ _]
      timeout: _ -> [_ _]
      tunnel: w2288 -> [w2292 _]
      event Mouse Down {
        n1577 = event-data() -> ("Time"=w2294:u32, "Coords"=w2293:T7, "Button"=w2295:u16)  [unwired: 6 out]
        n1578 = case shown="3" w2295 {
          tunnel: w2294 -> [_ _ w2401]
          tunnel: w2293 -> [_ w2332 w2399]
          tunnel: w2292 -> [_ _ w2397]
          frame 0, Default {
          }
          frame 1 {
            n1579 = property on="APD 2" class="ImageControl"() -> ("Displayed Image Position"=w2302:cluster{"Left":i32, "Top":i32})  [unwired: 2 in, 2 out]
            n1580 = property on="APD 1" class="ImageControl"() -> ("Displayed Image Position"=w2331:cluster{"Left":i32, "Top":i32})  [unwired: 2 in, 2 out]
            n1581 = property on="Detection Laser X" class="ImageControl"() -> ("Displayed Image Position"=w2328:cluster{"Left":i32, "Top":i32})  [unwired: 2 in, 2 out]
            n1582 = property on="Detection Laser Y" class="ImageControl"() -> ("Displayed Image Position"=w2327:cluster{"Left":i32, "Top":i32})  [unwired: 2 in, 2 out]
            n1583 = property on="APD 2" class="ImageControl"() -> ("Displayed Image Size"=w2301:cluster{"Width":u32, "Height":u32})  [unwired: 2 in, 2 out]
            n1584 = property on="APD 1" class="ImageControl"() -> ("Displayed Image Size"=w2329:cluster{"Width":u32, "Height":u32})  [unwired: 2 in, 2 out]
            n1585 = property on="Detection Laser X" class="ImageControl"() -> ("Displayed Image Size"=w2330:cluster{"Width":u32, "Height":u32})  [unwired: 2 in, 2 out]
            n1586 = property on="Detection Laser Y" class="ImageControl"() -> ("Displayed Image Size"=w2326:cluster{"Width":u32, "Height":u32})  [unwired: 2 in, 2 out]
            n1587 = Unbundle By Name(w2301) -> ("Width"=w2298:u32, "Height"=w2297:u32)
            n1588 = Unbundle By Name(w2302) -> ("Left"=w2300:i32, "Top"=w2299:i32)
            n1589 = Unbundle By Name(w2329) -> ("Width"=w2323:u32, "Height"=w2322:u32)
            n1590 = Unbundle By Name(w2330) -> ("Width"=w2319:u32, "Height"=w2318:u32)
            n1591 = Unbundle By Name(w2326) -> ("Width"=w2315:u32, "Height"=w2314:u32)
            n1592 = Unbundle By Name(w2331) -> ("Left"=w2325:i32, "Top"=w2324:i32)
            n1593 = Unbundle By Name(w2328) -> ("Left"=w2321:i32, "Top"=w2320:i32)
            n1594 = Unbundle By Name(w2327) -> ("Left"=w2317:i32, "Top"=w2316:i32)
            n1595 = Bundle("Left"=w2300, "Top"=w2299, "Width"=w2298, "Height"=w2297) -> (w2296:T31)  [unwired: 1 in]
            n1596 = Bundle("Left"=w2325, "Top"=w2324, "Width"=w2323, "Height"=w2322) -> (w2313:T31)  [unwired: 1 in]
            n1597 = Bundle("Left"=w2321, "Top"=w2320, "Width"=w2319, "Height"=w2318) -> (w2312:T31)  [unwired: 1 in]
            n1598 = Bundle("Left"=w2317, "Top"=w2316, "Width"=w2315, "Height"=w2314) -> (w2311:T31)  [unwired: 1 in]
            n1599 = Build Cluster Array(w2296, w2313, w2312, w2311) -> (w2310:T32)
            n1600 = for {
              tunnel: w2332 -> [w2343]
              tunnel: w2310 -> [w2344] mode=indexing
              shift-right: [w2341] -> w2308
              shift-left: TRUE -> [w2342]
              shift-right: [w2340] -> w2306
              shift-left: _ -> [w2336]
              shift-right: [w2339] -> w2305
              shift-left: _ -> [w2335]
              shift-right: [w2338] -> w2304
              shift-left: _ -> [w2334]
              shift-right: [w2337] -> w2303
              shift-left: _ -> [w2333]
              n1601 = case shown="True" w2342 {
                selector: w2342 -> [w2349 _]
                tunnel: w2344 -> [_ w2358]
                tunnel: w2343 -> [_ w2356]
                tunnel: [w2349 w2354] -> w2341
                tunnel: [w2348 w2353] -> w2340
                tunnel: [w2347 w2352] -> w2339
                tunnel: [w2346 w2351] -> w2338
                tunnel: [w2345 w2350] -> w2337
                tunnel: w2336 -> [w2348 _]
                tunnel: w2335 -> [w2347 _]
                tunnel: w2334 -> [w2346 _]
                tunnel: w2333 -> [w2345 _]
                frame False {
                }
                frame True {
                  n1602 = Unbundle(w2358) -> (w2357:T31)
                  n1603 = call "isclickinwindow.vi"("Image Param"=w2357, "Point32"=w2356) -> ("4 Y"=w2350:i32, "3 Height"=w2351:i32, "2 X"=w2352:i32, "1 Width"=w2353:i32, "In image?"=w2355:bool)  [unwired: 1 in]
                  n1604 = Not(x=w2355) -> (.not. x?=w2354:bool)
                }
              }
            }
            n1605 = Not(x=w2308) -> (.not. x?=w2307:bool)
            n1606 = case shown="True" w2307 {
              tunnel: w2305 -> [_ w2372]
              tunnel: w2303 -> [_ w2371]
              tunnel: w2306 -> [_ w2370]
              tunnel: w2304 -> [_ w2369]
              frame False {
              }
              frame True {
                w2359 = FALSE ("Get Point")
                n1607 = local read "Scan lines (y)"() -> (w2374:u64)
                n1608 = disable-structure shown="Disabled" {
                  frame Disabled {
                  }
                  frame Enabled {
                  }
                }
                n1609 = local read "Actual MCL Inc (V)"() -> (w2368:dbl)
                n1610 = local read "Scan steps (MCL)"() -> (w2373:u64)
                n1611 = Divide "Y Pix/step"(x=w2369, y=w2374) -> (x/y=w2381:dbl)
                n1612 = Divide "Y V/pix"(x=w2368, y=w2381) -> (x/y=w2380:dbl)
                n1613 = Divide "Y half step offset"(x=w2368, y=2.0) -> (x/y=w2382:dbl)
                n1614 = Divide "X pix/step"(x=w2370, y=w2373) -> (x/y=w2379:dbl)
                n1615 = Negate(x=w2382) -> (-x=w2383:dbl)
                n1616 = local read "Initial Y"() -> (w2389:dbl)
                n1617 = Multiply(x=w2371, y=w2380) -> (x*y=w2390:dbl)
                n1618 = Divide "X half step offset"(x=w2368, y=2.0) -> (x/y=w2376:dbl)
                n1619 = Divide "X V/pix"(x=w2368, y=w2379) -> (x/y=w2378:dbl)
                n1620 = Multiply(x=w2368, y=w2373) -> (x*y=w2385:dbl)
                n1621 = Compound Arithmetic op=ADD(w2383, w2390, w2389) -> (w2360:dbl)
                "Pointer Y (V)" <- w2360
                n1622 = Multiply(x=w2378, y=w2372) -> (x*y=w2387:dbl)
                n1623 = Negate(x=w2376) -> (-x=w2375:dbl)
                n1624 = local read "Initial X"() -> (w2388:dbl)
                n1625 = Negate(x=w2387) -> (-x=w2386:dbl)
                n1626 = Compound Arithmetic op=ADD(w2375, w2385, w2388, w2386) -> (w2361:dbl)
                "Pointer X (V)" <- w2361
                n1627 = case shown="True" "Set High F Confocal Spot (X-Y)" {
                  tunnel: w2361 -> [_ w2391]
                  tunnel: w2360 -> [_ w2392]
                  frame False {
                  }
                  frame True {
                    "Confocal Y 2 (V)" <- w2392
                    "Confocal X 2 (V)" <- w2391
                  }
                }
                n1628 = Or(x="Set X Only", y="Set Confocal Spot (X-Y)") -> (x .or. y?=w2364:bool)
                n1629 = Or(x="Set Confocal Spot (X-Y)", y="Set Y Only") -> (x .or. y?=w2363:bool)
                n1630 = case shown="True" w2364 {
                  tunnel: w2361 -> [_ w2393]
                  frame False {
                  }
                  frame True {
                    n1631 = property on="AO2" class="Slide (strict)"("Val(Sgnl)"=w2393) -> ()  [unwired: 2 in, 2 out]
                    "Confocal X 1 (V)" <- w2393
                  }
                }
                n1632 = case shown="True" w2363 {
                  tunnel: w2360 -> [_ w2394]
                  frame False {
                  }
                  frame True {
                    n1633 = property on="AO1" class="Slide (strict)"("Val(Sgnl)"=w2394) -> ()  [unwired: 2 in, 2 out]
                    "Confocal Y 1 (V)" <- w2394
                  }
                }
                n1634 = local write "Set High F Confocal Spot (X-Y)"(w2359) -> ()